vi "UHR-Fleezers Control (host) - 12.8.1.vi"() -> ()   [LabVIEW 2012] (continued)
                                n2135 = Greater?(x=w3246, y=70.0) -> (0:w3244:bool)
                                n2136 = property on="Remove Action Offset" class="Bool (strict)"("Val(Sgnl)"=w3244) -> ()  [unwired: 2 in, 2 out]
                                }
                                }
                                }
                                }
                                frame #4 {
                                n2137 = Wait (ms)(milliseconds to wait=u32 500) -> ()  [unwired: 1 out]
                                }
                                frame #5 {
                                n2138 = local read "Mean"() -> (w3255:dbl)
                                n2139 = Greater?(x=w3255, y=11.0) -> (0:w3249:bool)
                                n2140 = Not(x=w3249) -> (.not. x?=w3250:bool)
                                n2141 = And(x=w3250, y="Shift confocal") -> (x .and. y?=w3252:bool)
                                n2142 = And(x=w3249, y="Shift confocal") -> (x .and. y?=w3253:bool)
                                n2143 = case shown="True" w3253 {
                                frame False {
                                }
                                frame True {
                                n2144 = local read "Confocal Y 2 (V)"() -> (w3259:dbl)
                                n2145 = local read "Confocal X 2 (V)"() -> (w3258:dbl)
                                n2146 = property on="AO1" class="Slide (strict)"("Val(Sgnl)"=w3259) -> ()  [unwired: 2 in, 2 out]
                                n2147 = property on="AO2" class="Slide (strict)"("Val(Sgnl)"=w3258) -> ()  [unwired: 2 in, 2 out]
                                }
                                }
                                n2148 = case shown="True" w3252 {
                                frame False {
                                }
                                frame True {
                                n2149 = local read "Confocal Y 1 (V)"() -> (w3257:dbl)
                                n2150 = local read "Confocal X 1 (V)"() -> (w3256:dbl)
                                n2151 = property on="AO1" class="Slide (strict)"("Val(Sgnl)"=w3257) -> ()  [unwired: 2 in, 2 out]
                                n2152 = property on="AO2" class="Slide (strict)"("Val(Sgnl)"=w3256) -> ()  [unwired: 2 in, 2 out]
                                }
                                }
                                }
                                frame #6 {
                                n2153 = Wait (ms)(milliseconds to wait=u32 1500) -> ()  [unwired: 1 out]
                                }
                                frame #7 {
                                n2154 = property on="Rem fb disp offset" class="Bool (strict)"("Val(Sgnl)"=TRUE ("Value (Signaling)")) -> ()  [unwired: 2 in, 2 out]
                                }
                                }
                                }
                                frame True {
                                n2155 = flat-sequence {
                                tunnel: w3262 -> [w3263]
                                frame #0 {
                                n2156 = property on="Trap Delta (MHz)" class="DigNum (strict)"("Val(Sgnl)"=w3263) -> ()  [unwired: 2 in, 2 out]
                                }
                                frame #1 {
                                n2157 = Wait (ms)(milliseconds to wait=u32 500) -> ()  [unwired: 1 out]
                                }
                                frame #2 {
                                n2158 = local read "Shift confocal"() -> (w3269:bool)
                                n2159 = local read "Mean"() -> (w3271:dbl)
                                n2160 = Greater?(x=w3271, y=11.0) -> (0:w3268:bool)
                                n2161 = Not(x=w3268) -> (.not. x?=w3267:bool)
                                n2162 = And(x=w3267, y=w3269) -> (x .and. y?=w3265:bool)
                                n2163 = And(x=w3268, y=w3269) -> (x .and. y?=w3266:bool)
                                n2164 = case shown="True" w3266 {
                                frame False {
                                }
                                frame True {
                                n2165 = local read "Confocal Y 2 (V)"() -> (w3275:dbl)
                                n2166 = local read "Confocal X 2 (V)"() -> (w3274:dbl)
                                n2167 = property on="AO2" class="Slide (strict)"("Val(Sgnl)"=w3274) -> ()  [unwired: 2 in, 2 out]
                                n2168 = property on="AO1" class="Slide (strict)"("Val(Sgnl)"=w3275) -> ()  [unwired: 2 in, 2 out]
                                }
                                }
                                n2169 = case shown="True" w3265 {
                                frame False {
                                }
                                frame True {
                                n2170 = local read "Confocal X 1 (V)"() -> (w3272:dbl)
                                n2171 = local read "Confocal Y 1 (V)"() -> (w3273:dbl)
                                n2172 = property on="AO2" class="Slide (strict)"("Val(Sgnl)"=w3272) -> ()  [unwired: 2 in, 2 out]
                                n2173 = property on="AO1" class="Slide (strict)"("Val(Sgnl)"=w3273) -> ()  [unwired: 2 in, 2 out]
                                }
                                }
                                }
                                }
                                }
                                }
                                }
                                }
                                }
                                frame "Image" {
                                n2174 = property on="Confocal Image" class="Bool (strict)"("Val(Sgnl)"=TRUE ("Value (Signaling)")) -> ()  [unwired: 2 in, 2 out]
                                }
                              }
                              n2175 = local write "Fl. High"(FALSE ("Fl. High")) -> ()
                              n2176 = local read "Time (s)"() -> (w3209:dbl)
                            }
                            frame #1 {
                              n2177 = case shown="True" "Auto F Reset" {
                                tunnel: w3281 -> [_ w3286]
                                tunnel: w3280 -> [_ w3285]
                                tunnel: w3279 -> [_ w3284]
                                tunnel: w3278 -> [_ w3283]
                                frame False {
                                }
                                frame True {
                                n2178 = node-c288() -> (w3288:T27)  [unwired: 4 in]
                                n2179 = timed-loop {
                                timing: w3288 -> [_]
                                timing-out: [_] -> w3287
                                tunnel: w3286 -> [w3293]
                                tunnel: w3285 -> [w3292]
                                tunnel: w3284 -> [w3291]
                                tunnel: w3283 -> [w3290]
                                stop <- w3289 stop-if-true
                                n2180 = node-c288() -> ()  [unwired: 1 in, 1 out]
                                n2181 = local read "Fl. Delta Thresh. (kHz)"() -> (w3302:dbl)
                                n2182 = local read "APD to Watch"() -> (w3303:bool)
                                n2183 = local read "Delta Fl. 1"() -> (w3304:dbl)
                                n2184 = local read "Delta Fl. 2"() -> (w3305:dbl)
                                n2185 = local read "Fl. Triggered..."() -> (w3296:bool)
                                n2186 = local read "Stop All"() -> (w3297:bool)
                                n2187 = local read "Reset Force"() -> (w3295:bool)
                                n2188 = Multiply(x=w3302, y=1000.0) -> (x*y=w3300:dbl)
                                n2189 = Select(t=w3304, s=w3303, f=w3305) -> (s? t:f=w3299:dbl)
                                n2190 = Not(x=w3296) -> (.not. x?=w3294:bool)
                                n2191 = Greater?(x=w3299, y=w3300) -> (0:w3298:bool)
                                n2192 = Compound Arithmetic op=OR(w3298, w3297, w3294, w3295) -> (w3289:bool)
                                n2193 = case shown="True" w3289 {
                                tunnel: w3293 -> [_ w3309]
                                tunnel: w3292 -> [_ w3313]
                                tunnel: w3291 -> [_ w3312]
                                tunnel: w3290 -> [_ w3311]
                                frame False {
                                }
                                frame True {
                                n2194 = case shown="\"Yank\"" w3313 {
                                tunnel: w3312 -> [_ w3323]
                                tunnel: w3311 -> [_ w3321]
                                frame "Image", Default {
                                }
                                frame "Yank" {
                                n2195 = flat-sequence {
                                tunnel: [w3326] -> w3324
                                tunnel: w3323 -> [w3326]
                                tunnel: [w3325] -> w3322
                                tunnel: w3321 -> [w3325]
                                tunnel: w3324 -> [w3332]
                                tunnel: w3322 -> [w3330]
                                frame #0 {
                                n2196 = local read "Yank Delay (s)"() -> (w3329:dbl)
                                n2197 = Multiply(x=w3329, y=1000.0) -> (x*y=w3327:dbl)
                                n2198 = Wait (ms)(milliseconds to wait=w3327) -> ()  [unwired: 1 out]
                                }
                                frame #1 {
                                n2199 = local read "Yank to which?"() -> (w3331:bool)
                                n2200 = case shown="False" w3331 {
                                tunnel: w3332 -> [_ w3360]
                                tunnel: w3330 -> [w3333 _]
                                frame False {
                                n2201 = flat-sequence {
                                tunnel: w3333 -> [w3334]
                                frame #0 {
                                n2202 = property on="Trap Pos FB SP" class="DigNum (strict)"("Val(Sgnl)"=w3334) -> ()  [unwired: 2 in, 2 out]
                                }
                                frame #1 {
                                n2203 = Wait (ms)(milliseconds to wait=u32 700) -> ()  [unwired: 1 out]
                                }
                                frame #2 {
                                n2204 = local read "Action (%)"() -> (w3339:dbl)
                                n2205 = Absolute Value(x=w3339) -> (abs(x)=w3338:dbl)
                                n2206 = Greater?(x=w3338, y=70.0) -> (0:w3336:bool)
                                n2207 = property on="Remove Action Offset" class="Bool (strict)"("Val(Sgnl)"=w3336) -> ()  [unwired: 2 in, 2 out]
                                }
                                frame #3 {
                                n2208 = for {
                                N: 4 -> [_]
                                n2209 = flat-sequence {
                                frame #0 {
                                n2210 = Wait (ms)(milliseconds to wait=u32 500) -> ()  [unwired: 1 out]
                                }
                                frame #1 {
                                n2211 = local read "Action (%)"() -> (w3345:dbl)
                                n2212 = Absolute Value(x=w3345) -> (abs(x)=w3344:dbl)
                                n2213 = Greater?(x=w3344, y=70.0) -> (0:w3342:bool)
                                n2214 = property on="Remove Action Offset" class="Bool (strict)"("Val(Sgnl)"=w3342) -> ()  [unwired: 2 in, 2 out]
                                }
                                }
                                }
                                }
                                frame #4 {
                                n2215 = Wait (ms)(milliseconds to wait=u32 500) -> ()  [unwired: 1 out]
                                }
                                frame #5 {
                                n2216 = local read "Shift confocal"() -> (w3350:bool)
                                n2217 = local read "Mean"() -> (w3353:dbl)
                                n2218 = Greater?(x=w3353, y=11.0) -> (0:w3349:bool)
                                n2219 = Not(x=w3349) -> (.not. x?=w3348:bool)
                                n2220 = And(x=w3349, y=w3350) -> (x .and. y?=w3351:bool)
                                n2221 = And(x=w3348, y=w3350) -> (x .and. y?=w3347:bool)
                                n2222 = case shown="True" w3351 {
                                frame False {
                                }
                                frame True {
                                n2223 = local read "Confocal X 2 (V)"() -> (w3356:dbl)
                                n2224 = local read "Confocal Y 2 (V)"() -> (w3357:dbl)
                                n2225 = property on="AO2" class="Slide (strict)"("Val(Sgnl)"=w3356) -> ()  [unwired: 2 in, 2 out]
                                n2226 = property on="AO1" class="Slide (strict)"("Val(Sgnl)"=w3357) -> ()  [unwired: 2 in, 2 out]
                                }
                                }
                                n2227 = case shown="True" w3347 {
                                frame False {
                                }
                                frame True {
                                n2228 = local read "Confocal Y 1 (V)"() -> (w3355:dbl)
                                n2229 = local read "Confocal X 1 (V)"() -> (w3354:dbl)
                                n2230 = property on="AO1" class="Slide (strict)"("Val(Sgnl)"=w3355) -> ()  [unwired: 2 in, 2 out]
                                n2231 = property on="AO2" class="Slide (strict)"("Val(Sgnl)"=w3354) -> ()  [unwired: 2 in, 2 out]
                                }
                                }
                                }
                                frame #6 {
                                n2232 = Wait (ms)(milliseconds to wait=u32 1500) -> ()  [unwired: 1 out]
                                }
                                frame #7 {
                                n2233 = property on="Rem fb disp offset" class="Bool (strict)"("Val(Sgnl)"=TRUE ("Value (Signaling)")) -> ()  [unwired: 2 in, 2 out]
                                }
                                }
                                }
                                frame True {
                                n2234 = flat-sequence {
                                tunnel: w3360 -> [w3361]
                                frame #0 {
                                n2235 = property on="Trap Delta (MHz)" class="DigNum (strict)"("Val(Sgnl)"=w3361) -> ()  [unwired: 2 in, 2 out]
                                }
                                frame #1 {
                                n2236 = Wait (ms)(milliseconds to wait=u32 500) -> ()  [unwired: 1 out]
                                }
                                frame #2 {
                                n2237 = local read "Shift confocal"() -> (w3367:bool)
                                n2238 = local read "Mean"() -> (w3368:dbl)
                                n2239 = Greater?(x=w3368, y=11.0) -> (0:w3366:bool)
                                n2240 = And(x=w3366, y=w3367) -> (x .and. y?=w3364:bool)
                                n2241 = Not(x=w3366) -> (.not. x?=w3365:bool)
                                n2242 = And(x=w3365, y=w3367) -> (x .and. y?=w3363:bool)
                                n2243 = case shown="True" w3364 {
                                frame False {
                                }
                                frame True {
                                n2244 = local read "Confocal Y 2 (V)"() -> (w3373:dbl)
                                n2245 = local read "Confocal X 2 (V)"() -> (w3372:dbl)
                                n2246 = property on="AO1" class="Slide (strict)"("Val(Sgnl)"=w3373) -> ()  [unwired: 2 in, 2 out]
                                n2247 = property on="AO2" class="Slide (strict)"("Val(Sgnl)"=w3372) -> ()  [unwired: 2 in, 2 out]
                                }
                                }
                                n2248 = case shown="True" w3363 {
                                frame False {
                                }
                                frame True {
                                n2249 = local read "Confocal Y 1 (V)"() -> (w3371:dbl)
                                n2250 = local read "Confocal X 1 (V)"() -> (w3370:dbl)
                                n2251 = property on="AO2" class="Slide (strict)"("Val(Sgnl)"=w3370) -> ()  [unwired: 2 in, 2 out]
                                n2252 = property on="AO1" class="Slide (strict)"("Val(Sgnl)"=w3371) -> ()  [unwired: 2 in, 2 out]
                                }
                                }
                                }
                                }
                                }
                                }
                                }
                                }
                                }
                                }
                                n2253 = local read "Time (s)"() -> (w3308:dbl)
                                n2254 = Subtract(x=w3309, y=w3308) -> (x-y=w3320:dbl)
                                n2255 = Number To Decimal String(number=w3320, width (-)=i16 0) -> (decimal integer string=w3318:string)
                                n2256 = Concatenate Strings(w3318, " s fluorescence event") -> (w3315:string)
                                n2257 = local read "Messages"() -> (w3316:string)
                                n2258 = local write "Duration (s)"(w3320) -> ()
                                n2259 = call "Update messages.vi"("Message to add"=w3315, "Old message string"=w3316) -> ("New message string"=w3314:string)
                                n2260 = local write "Messages"(w3314) -> ()
                                n2261 = call <vilib>:"Beep.vi"() -> ()  [unwired: 12 in]
                                n2262 = local write "Reset Force"(FALSE ("Force Reset")) -> ()
                                n2263 = local write "Fl. High"(TRUE ("Fl. High")) -> ()
                                n2264 = local write "Waiting"(TRUE ("Waiting")) -> ()
                                }
                                }
                                n2265 = node-c288() -> ()  [unwired: 1 in, 1 out]
                                }
                                n2266 = node-c288(w3287) -> ()  [unwired: 1 out]
                                }
                              }
                            }
                          }
                          n2267 = local read "Trap Delta (MHz)"() -> (w3199:dbl)
                          n2268 = local read "Trap Pos FB SP"() -> (w3197:fxp<+/-,16,1>)
                        }
                      }
                    }
                    frame True {
                      n2269 = flat-sequence {
                        tunnel: w3384 -> [w3394]
                        tunnel: [w3394] -> w3388
                        tunnel: w3387 -> [w3393]
                        tunnel: [w3393] -> w3386
                        tunnel: [w3392] -> w3385
                        tunnel: w3383 -> [w3391]
                        tunnel: [w3390] -> w3382
                        tunnel: w3379 -> [w3389]
                        tunnel: [w3389] -> w3378
                        tunnel: w3388 -> [w3464]
                        tunnel: w3386 -> [w3463]
                        tunnel: w3385 -> [w3462]
                        tunnel: w3382 -> [w3461]
                        tunnel: w3378 -> [w3460]
                        tunnel: [w3461] -> w3381
                        frame #0 {
                          n2270 = call <vilib>:"Beep.vi"() -> ()  [unwired: 3 in, 9 out]
                          n2271 = local write "Waiting"(FALSE ("Waiting")) -> ()
                          n2272 = Increment(x=w3391) -> (x+1=w3390:u8)
                          n2273 = case shown="\"Yank\"" w3393 {
                            tunnel: w3390 -> [_ _ w3400]
                            frame "Image" {
                              n2274 = property on="Confocal Image" class="Bool (strict)"("Val(Sgnl)"=TRUE ("Value (Signaling)")) -> ()  [unwired: 2 in, 2 out]
                            }
                            frame "Alarm", Default {
                            }
                            frame "Yank" {
                              n2275 = flat-sequence {
                                tunnel: w3400 -> [w3403]
                                tunnel: [w3402] -> w3399
                                tunnel: ["N Array El"] -> w3398
                                tunnel: w3399 -> [w3417]
                                tunnel: w3398 -> [w3413]
                                frame #0 {
                                n2276 = Multiply(x="Yank Delay (s)", y=1000.0) -> (x*y=w3406:dbl)
                                n2277 = Quotient & Remainder(x=w3403, y="N Array El") -> (x-y*floor(x/y)=w3402:u8)  [unwired: 1 out]
                                n2278 = Wait (ms)(milliseconds to wait=w3406) -> ()  [unwired: 1 out]
                                }
                                frame #1 {
                                n2279 = Random Number (0-1)() -> (number: 0 to 1=w3414:dbl)
                                n2280 = Multiply(x=w3413, y=w3414) -> (x*y=w3412:dbl)
                                n2281 = Round Toward -Infinity(1:w3412) -> (0:w3411:dbl)
                                n2282 = Select(t=w3411, s="Random Choice", f=w3417) -> (s? t:f=w3415:dbl)
                                n2283 = Select(t="Yank to Trap Delta (MHz)", s="Yank to which?", f="Yank to SP") -> (s? t:f=w3408:dbl[])
                                n2284 = Index Array(array=w3408, index=w3415) -> (element=w3418:dbl)
                                n2285 = case shown="False" "Yank to which?" {
                                tunnel: w3418 -> [w3419 w3445]
                                frame False {
                                n2286 = flat-sequence {
                                tunnel: w3419 -> [w3420]
                                frame #0 {
                                n2287 = property on="Trap Pos FB SP" class="DigNum (strict)"("Val(Sgnl)"=w3420) -> ()  [unwired: 2 in, 2 out]
                                }
                                frame #1 {
                                n2288 = Wait (ms)(milliseconds to wait=u32 700) -> ()  [unwired: 1 out]
                                }
                                frame #2 {
                                n2289 = local read "Action (%)"() -> (w3425:dbl)
                                n2290 = Absolute Value(x=w3425) -> (abs(x)=w3424:dbl)
                                n2291 = Greater?(x=w3424, y=70.0) -> (0:w3422:bool)
                                n2292 = property on="Remove Action Offset" class="Bool (strict)"("Val(Sgnl)"=w3422) -> ()  [unwired: 2 in, 2 out]
                                }
                                frame #3 {
                                n2293 = for {
                                N: 4 -> [_]
                                n2294 = flat-sequence {
                                frame #0 {
                                n2295 = Wait (ms)(milliseconds to wait=u32 500) -> ()  [unwired: 1 out]
                                }
                                frame #1 {
                                n2296 = local read "Action (%)"() -> (w3431:dbl)
                                n2297 = Absolute Value(x=w3431) -> (abs(x)=w3430:dbl)
                                n2298 = Greater?(x=w3430, y=70.0) -> (0:w3428:bool)
                                n2299 = property on="Remove Action Offset" class="Bool (strict)"("Val(Sgnl)"=w3428) -> ()  [unwired: 2 in, 2 out]
                                }
                                }
                                }
                                }
                                frame #4 {
                                n2300 = local read "Shift confocal"() -> (w3435:bool)
                                n2301 = local read "Mean"() -> (w3438:dbl)
                                n2302 = Greater?(x=w3438, y=11.0) -> (0:w3434:bool)
                                n2303 = Not(x=w3434) -> (.not. x?=w3433:bool)
                                n2304 = And(x=w3433, y=w3435) -> (x .and. y?=w3432:bool)
                                n2305 = And(x=w3434, y=w3435) -> (x .and. y?=w3436:bool)
                                n2306 = case shown="True" w3436 {
                                frame False {
                                }
                                frame True {
                                n2307 = local read "Confocal X 2 (V)"() -> (w3441:dbl)
                                n2308 = local read "Confocal Y 2 (V)"() -> (w3442:dbl)
                                n2309 = property on="AO2" class="Slide (strict)"("Val(Sgnl)"=w3441) -> ()  [unwired: 2 in, 2 out]
                                n2310 = property on="AO1" class="Slide (strict)"("Val(Sgnl)"=w3442) -> ()  [unwired: 2 in, 2 out]
                                }
                                }
                                n2311 = case shown="True" w3432 {
                                frame False {
                                }
                                frame True {
                                n2312 = local read "Confocal X 1 (V)"() -> (w3439:dbl)
                                n2313 = local read "Confocal Y 1 (V)"() -> (w3440:dbl)
                                n2314 = property on="AO1" class="Slide (strict)"("Val(Sgnl)"=w3440) -> ()  [unwired: 2 in, 2 out]
                                n2315 = property on="AO2" class="Slide (strict)"("Val(Sgnl)"=w3439) -> ()  [unwired: 2 in, 2 out]
                                }
                                }
                                }
                                frame #5 {
                                n2316 = Wait (ms)(milliseconds to wait=u32 1500) -> ()  [unwired: 1 out]
                                }
                                frame #6 {
                                n2317 = property on="Rem fb disp offset" class="Bool (strict)"("Val(Sgnl)"=TRUE ("Value (Signaling)")) -> ()  [unwired: 2 in, 2 out]
                                }
                                }
                                }
                                frame True {
                                n2318 = flat-sequence {
                                tunnel: w3445 -> [w3446]
                                frame #0 {
                                n2319 = property on="Trap Delta (MHz)" class="DigNum (strict)"("Val(Sgnl)"=w3446) -> ()  [unwired: 2 in, 2 out]
                                }
                                frame #1 {
                                n2320 = Wait (ms)(milliseconds to wait=u32 500) -> ()  [unwired: 1 out]
                                }
                                frame #2 {
                                n2321 = local read "Shift confocal"() -> (w3450:bool)
                                n2322 = local read "Mean"() -> (w3448:dbl)
                                n2323 = Greater?(x=w3448, y=11.0) -> (0:w3451:bool)
                                n2324 = Not(x=w3451) -> (.not. x?=w3452:bool)
                                n2325 = And(x=w3452, y=w3450) -> (x .and. y?=w3454:bool)
                                n2326 = And(x=w3451, y=w3450) -> (x .and. y?=w3453:bool)
                                n2327 = case shown="True" w3453 {
                                frame False {
                                }
                                frame True {
                                n2328 = local read "Confocal Y 2 (V)"() -> (w3458:dbl)
                                n2329 = local read "Confocal X 2 (V)"() -> (w3457:dbl)
                                n2330 = property on="AO1" class="Slide (strict)"("Val(Sgnl)"=w3458) -> ()  [unwired: 2 in, 2 out]
                                n2331 = property on="AO2" class="Slide (strict)"("Val(Sgnl)"=w3457) -> ()  [unwired: 2 in, 2 out]
                                }
                                }
                                n2332 = case shown="True" w3454 {
                                frame False {
                                }
                                frame True {
                                n2333 = local read "Confocal X 1 (V)"() -> (w3455:dbl)
                                n2334 = local read "Confocal Y 1 (V)"() -> (w3456:dbl)
                                n2335 = property on="AO2" class="Slide (strict)"("Val(Sgnl)"=w3455) -> ()  [unwired: 2 in, 2 out]
                                n2336 = property on="AO1" class="Slide (strict)"("Val(Sgnl)"=w3456) -> ()  [unwired: 2 in, 2 out]
                                }
                                }
                                }
                                }
                                }
                                }
                                }
                              }
                            }
                          }
                          n2337 = local read "Time (s)"() -> (w3392:dbl)
                          "Fl. High" <- TRUE ("Yanking")
                        }
                        frame #1 {
                          n2338 = local read "Auto F Reset"() -> (w3459:bool)
                          n2339 = case shown="True" w3459 {
                            tunnel: w3464 -> [_ w3468]
                            tunnel: w3463 -> [_ w3467]
                            tunnel: w3462 -> [_ w3466]
                            tunnel: w3460 -> [_ w3465]
                            frame False {
                            }
                            frame True {
                              n2340 = node-c288() -> (w3470:T27)  [unwired: 4 out]
                              n2341 = timed-loop {
                                timing: w3470 -> [_]
                                timing-out: [_] -> w3469
                                tunnel: w3468 -> [w3488]
                                tunnel: w3467 -> [w3487]
                                tunnel: w3466 -> [w3486]
                                tunnel: w3465 -> [w3485]
                                stop <- w3471 stop-if-true
                                n2342 = node-c288() -> ()  [unwired: 2 out]
                                n2343 = local read "Fl. Delta Thresh. (kHz)"() -> (w3479:dbl)
                                n2344 = local read "Fl. Triggered..."() -> (w3484:bool)
                                n2345 = local read "Delta Fl. 1"() -> (w3475:dbl)
                                n2346 = local read "Delta Fl. 2"() -> (w3473:dbl)
                                n2347 = local read "Stop All"() -> (w3482:bool)
                                n2348 = local read "APD to Watch"() -> (w3474:bool)
                                n2349 = Select(t=w3475, s=w3474, f=w3473) -> (s? t:f=w3472:dbl)
                                n2350 = Not(x=w3484) -> (.not. x?=w3483:bool)
                                n2351 = Multiply(x=w3479, y=1000.0) -> (x*y=w3478:dbl)
                                n2352 = Negate(x=w3478) -> (-x=w3477:dbl)
                                n2353 = Less?(x=w3472, y=w3477) -> (x < y?=w3481:bool)
                                n2354 = Compound Arithmetic op=OR(w3481, w3482, w3483, "Reset Force") -> (w3471:bool)
                                n2355 = case shown="True" w3471 {
                                tunnel: w3488 -> [_ w3503]
                                tunnel: w3487 -> [_ w3502]
                                tunnel: w3486 -> [_ w3492]
                                tunnel: w3485 -> [_ w3494]
                                frame False {
                                }
                                frame True {
                                n2356 = local read "Time (s)"() -> (w3493:dbl)
                                n2357 = case shown="\"Yank\"" w3502 {
                                tunnel: w3503 -> [_ w3506]
                                tunnel: w3494 -> [_ w3504]
                                frame "Image", Default {
                                }
                                frame "Yank" {
                                n2358 = flat-sequence {
                                tunnel: [w3512] -> w3507
                                tunnel: w3506 -> [w3512]
                                tunnel: [w3508] -> w3505
                                tunnel: w3504 -> [w3508]
                                tunnel: w3507 -> [w3515]
                                tunnel: w3505 -> [w3513]
                                frame #0 {
                                n2359 = local read "Yank Delay (s)"() -> (w3511:dbl)
                                n2360 = Multiply(x=w3511, y=1000.0) -> (x*y=w3509:dbl)
                                n2361 = Wait (ms)(milliseconds to wait=w3509) -> ()  [unwired: 1 out]
                                }
                                frame #1 {
                                n2362 = local read "Yank to which?"() -> (w3514:bool)
                                n2363 = case shown="False" w3514 {
                                tunnel: w3515 -> [_ w3542]
                                tunnel: w3513 -> [w3516 _]
                                frame False {
                                n2364 = flat-sequence {
                                tunnel: w3516 -> [w3517]
                                frame #0 {
                                n2365 = property on="Trap Pos FB SP" class="DigNum (strict)"("Val(Sgnl)"=w3517) -> ()  [unwired: 2 in, 2 out]
                                }
                                frame #1 {
                                n2366 = Wait (ms)(milliseconds to wait=u32 700) -> ()  [unwired: 1 out]
                                }
                                frame #2 {
                                n2367 = local read "Action (%)"() -> (w3522:dbl)
                                n2368 = Absolute Value(x=w3522) -> (abs(x)=w3521:dbl)
                                n2369 = Greater?(x=w3521, y=70.0) -> (0:w3519:bool)
                                n2370 = property on="Remove Action Offset" class="Bool (strict)"("Val(Sgnl)"=w3519) -> ()  [unwired: 2 in, 2 out]
                                }
                                frame #3 {
                                n2371 = for {
                                N: 4 -> [_]
                                n2372 = flat-sequence {
                                frame #0 {
                                n2373 = Wait (ms)(milliseconds to wait=u32 500) -> ()  [unwired: 1 out]
                                }
                                frame #1 {
                                n2374 = local read "Action (%)"() -> (w3528:dbl)
                                n2375 = Absolute Value(x=w3528) -> (abs(x)=w3527:dbl)
                                n2376 = Greater?(x=w3527, y=70.0) -> (0:w3525:bool)
                                n2377 = property on="Remove Action Offset" class="Bool (strict)"("Val(Sgnl)"=w3525) -> ()  [unwired: 2 in, 2 out]
                                }
                                }
                                }
                                }
                                frame #4 {
                                n2378 = local read "Shift confocal"() -> (w3533:bool)
                                n2379 = local read "Mean"() -> (w3535:dbl)
                                n2380 = Greater?(x=w3535, y=11.0) -> (0:w3532:bool)
                                n2381 = Not(x=w3532) -> (.not. x?=w3531:bool)
                                n2382 = And(x=w3532, y=w3533) -> (x .and. y?=w3530:bool)
                                n2383 = And(x=w3531, y=w3533) -> (x .and. y?=w3529:bool)
                                n2384 = case shown="True" w3530 {
                                frame False {
                                }
                                frame True {
                                n2385 = local read "Confocal Y 2 (V)"() -> (w3539:dbl)
                                n2386 = local read "Confocal X 2 (V)"() -> (w3538:dbl)
                                n2387 = property on="AO2" class="Slide (strict)"("Val(Sgnl)"=w3538) -> ()  [unwired: 2 in, 2 out]
                                n2388 = property on="AO1" class="Slide (strict)"("Val(Sgnl)"=w3539) -> ()  [unwired: 2 in, 2 out]
                                }
                                }
                                n2389 = case shown="True" w3529 {
                                frame False {
                                }
                                frame True {
                                n2390 = local read "Confocal X 1 (V)"() -> (w3536:dbl)
                                n2391 = local read "Confocal Y 1 (V)"() -> (w3537:dbl)
                                n2392 = property on="AO1" class="Slide (strict)"("Val(Sgnl)"=w3537) -> ()  [unwired: 2 in, 2 out]
                                n2393 = property on="AO2" class="Slide (strict)"("Val(Sgnl)"=w3536) -> ()  [unwired: 2 in, 2 out]
                                }
                                }
                                }
                                frame #5 {
                                n2394 = Wait (ms)(milliseconds to wait=u32 1500) -> ()  [unwired: 1 out]
                                }
                                frame #6 {
                                n2395 = property on="Rem fb disp offset" class="Bool (strict)"("Val(Sgnl)"=TRUE ("Value (Signaling)")) -> ()  [unwired: 2 in, 2 out]
                                }
                                }
                                }
                                frame True {
                                n2396 = flat-sequence {
                                tunnel: w3542 -> [w3543]
                                frame #0 {
                                n2397 = property on="Trap Delta (MHz)" class="DigNum (strict)"("Val(Sgnl)"=w3543) -> ()  [unwired: 2 in, 2 out]
                                }
                                frame #1 {
                                n2398 = Wait (ms)(milliseconds to wait=u32 500) -> ()  [unwired: 1 out]
                                }
                                frame #2 {
                                n2399 = local read "Shift confocal"() -> (w3549:bool)
                                n2400 = local read "Mean"() -> (w3551:dbl)
                                n2401 = Greater?(x=w3551, y=11.0) -> (0:w3548:bool)
                                n2402 = Not(x=w3548) -> (.not. x?=w3547:bool)
                                n2403 = And(x=w3548, y=w3549) -> (x .and. y?=w3546:bool)
                                n2404 = And(x=w3547, y=w3549) -> (x .and. y?=w3545:bool)
                                n2405 = case shown="True" w3546 {
                                frame False {
                                }
                                frame True {
                                n2406 = local read "Confocal Y 2 (V)"() -> (w3555:dbl)
                                n2407 = local read "Confocal X 2 (V)"() -> (w3554:dbl)
                                n2408 = property on="AO2" class="Slide (strict)"("Val(Sgnl)"=w3554) -> ()  [unwired: 2 in, 2 out]
                                n2409 = property on="AO1" class="Slide (strict)"("Val(Sgnl)"=w3555) -> ()  [unwired: 2 in, 2 out]
                                }
                                }
                                n2410 = case shown="True" w3545 {
                                frame False {
                                }
                                frame True {
                                n2411 = local read "Confocal Y 1 (V)"() -> (w3553:dbl)
                                n2412 = local read "Confocal X 1 (V)"() -> (w3552:dbl)
                                n2413 = property on="AO2" class="Slide (strict)"("Val(Sgnl)"=w3552) -> ()  [unwired: 2 in, 2 out]
                                n2414 = property on="AO1" class="Slide (strict)"("Val(Sgnl)"=w3553) -> ()  [unwired: 2 in, 2 out]
                                }
                                }
                                }
                                }
                                }
                                }
                                }
                                }
                                }
                                }
                                n2415 = local read "Messages"() -> (w3501:string)
                                n2416 = Subtract(x=w3493, y=w3492) -> (x-y=w3499:dbl)
                                "Duration (s)" <- w3499
                                n2417 = Number To Decimal String(number=w3499, width (-)=i16 0) -> (decimal integer string=w3497:string)
                                n2418 = Concatenate Strings(w3497, " s fluorescence event." ("string")) -> (w3495:string)
                                n2419 = call "Update messages.vi"("Message to add"=w3495, "Old message string"=w3501) -> ("New message string"=w3500:string)
                                n2420 = local write "Reset Force"(FALSE ("Reset Force")) -> ()
                                n2421 = local write "Waiting"(TRUE ("Waiting")) -> ()
                                n2422 = local write "Messages"(w3500) -> ()
                                n2423 = local write "Fl. High"(FALSE ("Fl. High")) -> ()
                                n2424 = call <vilib>:"Beep.vi"() -> ()  [unwired: 3 in, 9 out]
                                }
                                }
                                n2425 = node-c288() -> ()  [unwired: 2 out]
                              }
                              n2426 = node-c288(w3469) -> ()  [unwired: 1 out]
                            }
                          }
                        }
                      }
                      n2427 = local read "Trap Delta (MHz)"() -> (w3384:dbl)
                      n2428 = local read "Trap Pos FB SP"() -> (w3379:fxp<+/-,16,1>)
                    }
                  }
                }
                frame #1 {
                  n2429 = local read "Stop All"() -> (w3565:bool)
                  n2430 = local read "Fl. Triggered..."() -> (w3563:bool)
                  n2431 = Not(x=w3563) -> (.not. x?=w3564:bool)
                  n2432 = Or(x=w3564, y=w3565) -> (x .or. y?=w3562:bool)
                }
              }
              n2433 = case shown="True" w3156 {
                frame False {
                }
                frame True {
                  n2434 = local read "Confocal Y 1 (V)"() -> (w3166:dbl)
                  n2435 = local read "Confocal X 1 (V)"() -> (w3165:dbl)
                  n2436 = property on="AO2" class="Slide (strict)"("Val(Sgnl)"=w3165) -> ()  [unwired: 2 in, 2 out]
                  n2437 = property on="AO1" class="Slide (strict)"("Val(Sgnl)"=w3166) -> ()  [unwired: 2 in, 2 out]
                }
              }
              n2438 = case shown="True" w3156 {
                frame False {
                }
                frame True {
                  w3164 = FALSE ("Fl. High")
                  n2439 = local write "Waiting"(w3164) -> ()
                  n2440 = local write "Fl. High"(w3164) -> ()
                }
              }
              n2441 = node-c288() -> ()  [unwired: 2 out]
            }
            n2442 = node-c288(w3154) -> ()  [unwired: 1 out]
          }
        }
      }
      event "Stop All": Value Change {
        n2443 = event-data() -> ()  [unwired: 7 out]
        n2444 = local read "Stop All"() -> (w3570:bool)
      }
    }
    n2445 = node-c288() -> ()  [unwired: 2 out]
  }
  n2446 = node-c288(i64 1 ("Period"), 1 ("Processor")) -> (w85:T27)  [unwired: 2 out]
  n2447 = node-c288(w33) -> ()  [unwired: 1 out]
  n2448 = node-c288(w77) -> ()  [unwired: 1 out]
  n2449 = node-c288(w79) -> ()  [unwired: 1 out]
  n2450 = property on="Saved trap pos" class="WFGraph (strict)"("Visible"=FALSE) -> ()  [unwired: 2 in, 2 out]
  n2451 = property on="Trap Delta Graph" class="WFGraph (strict)"("Visible"=TRUE) -> ()  [unwired: 2 in, 2 out]
  n2452 = node-c288(w65) -> ()  [unwired: 1 out]
  n2453 = local write "Trap pos"(FALSE ("Trap pos")) -> ()
  n2454 = Unbundle By Name("sound format") -> ("sample rate (S/s)"=w4:dbl)
  n2455 = call <vilib>:"Sound Output Configure.vi"("number of samples/ch"="number of samples/ch", "sample mode"="sample mode", "sound format"="sound format", "device ID"="device ID") -> ("task ID"=w8:T42)  [unwired: 6 in, 1 out]
  n2456 = local read "DMA Update Period (s)"() -> (w5:dbl)
  n2457 = Multiply(x=w5, y=w4) -> (x*y=w3:dbl)
  n2458 = for "Sound time base" {
    N: w3 -> [_]
    tunnel: [w3571] -> w6 mode=indexing
    i -> [w3571]
  }
  n2459 = Reciprocal(x=w4) -> (1/x=w2:dbl)
  n2460 = Multiply(x=w6, y=w2) -> (x*y=w1:dbl[])
  n2461 = timed-loop "Main data acquisition loop (get data, process data for display, and save data to disk)" {
    tunnel: w23 -> [w3887]
    tunnel: w22 -> [w3886]
    tunnel: [w3915] -> w92
    tunnel: [w3910] -> w91
    timing: w85 -> [_]
    timing-out: [_] -> w84
    tunnel: w59 -> [w3771]
    tunnel: [w3597] -> w12
    tunnel: w8 -> [w3596]
    tunnel: w4 -> [w3594]
    tunnel: w3 -> [w3593]
    tunnel: w2 -> [w3592]
    tunnel: w1 -> [w3591]
    stop <- "Stop All" stop-if-true
    w3688 = "Initialize"
    # "List of channels in order (X or Y only):\nT1 X (mV)\nT2 X (mV)\nT1 X (nm)\nT2 X (nm)\nT1 FX (pN)\nT2 FX (pN)\nPosition Difference (nm)\nAPD1\nAPD2\nAPD3"
    # "T2 sum"
    # "T1 sum"
    # "Fluorescence data into FIFO for external control vi's\n(e.g., fluorescence triggering) - Duncan Nall"
    n2462 = node-c288() -> ()  [unwired: 2 out]
    n2463 = First Call?() -> (First Call?: T/F=w3723:bool)
    n2464 = Or(x="Reset", y=w3723) -> (x .or. y?=w3724:bool)
    n2465 = local read "Flushing P1"() -> (w3646:bool)
    n2466 = case "Reset data stream (manual reset or at begining of some rastering and imaging)" shown="True" w3724 {
      tunnel: w3887 -> [w4970 w4978]
      tunnel: w3886 -> [w4969 w4977]
      tunnel: [w4970 w4972] -> w3882
      tunnel: [w4969 w4971] -> w3881
      frame False {
      }
      frame True {
        w4975 = TRUE ("AI to FIFO")
        n2467 = local write "Overflow (data lost)"(FALSE ("Overflow (data lost)")) -> ()
        n2468 = call "reset FPGA DMA.vi"("error in"=w4977, "FPGA VI Reference In"=w4978) -> ("error out"=w4973:errorcluster, "FPGA VI Reference Out"=w4974:T24)
        n2469 = xnode "Read/Write Control"("FPGA VI Reference In"=w4974, "error in"=w4973, "AI to FIFO"=w4975, "APD to FIFO"=w4975) -> ("FPGA VI Reference Out"=w4972:T24, "error out"=w4971:errorcluster)
      }
    }
    n2470 = case shown="True" w3646 {
      frame False {
      }
      frame True {
        n2471 = local read "Flush rate (uL/m) P1"() -> (w4005:dbl)
        n2472 = local read "HP1 Flush Time (s)"() -> (w4014:dbl)
        n2473 = local read "DMA Update Period (s)"() -> (w4008:dbl)
        n2474 = Divide(x=w4005, y=60.0) -> (x/y=w4006:dbl)
        n2475 = Divide(x=w4014, y=w4008) -> (x/y=w4003:dbl)
        n2476 = feedback #4(0) -> (w4012:i32)
        n2477 = Increment(x=w4012) -> (x+1=w4002:i32)
        n2478 = Greater?(x=w4002, y=w4003) -> (0:w4011:bool)
        n2479 = Compound Arithmetic op=MULTIPLY(w4008, w4002, w4006) -> (→"P1 Flush Volume (uL)":dbl)
        n2480 = Divide(x=w4002, y=w4003) -> (x/y=→"P1 Flushing Bar":dbl)
        n2481 = case shown="True" w4011 {
          tunnel: w4002 -> [w4015 _]
          tunnel: [w4015 0] -> w4010
          frame False {
          }
          frame True {
            w4016 = FALSE ("Flushing P1")
            n2482 = local write "Inject Pump 1"(w4016) -> ()
            n2483 = local write "Flushing P1"(w4016) -> ()
            n2484 = property on="Clear Volume P1" class="Bool (strict)"("Val(Sgnl)"=TRUE ("Value (Signaling)")) -> ()  [unwired: 2 in, 2 out]
          }
        }
        n2485 = feedback-in #4(w4010) -> ()
      }
    }
    n2486 = Or(x="Start AOD Scan", y="Trap Raster Scan") -> (x .or. y?=w3846:bool)
    n2487 = case "Start AOM raster scan" shown="True" w3846 {
      tunnel: w3882 -> [w4820 w4830]
      tunnel: w3881 -> [w4819 w4829]
      tunnel: [w4820 w4823] -> w3880
      tunnel: [w4819 w4822] -> w3879
      frame False {
      }
      frame True {
        n2488 = case shown="True" "Restart DMA? (AOD)" {
          tunnel: [w4868 w4870] -> w4824
          tunnel: [w4867 w4869] -> w4825
          tunnel: w4830 -> [w4868 w4872]
          tunnel: w4829 -> [w4867 w4871]
          frame False {
          }
          frame True {
            n2489 = local write "Overflow (data lost)"(FALSE ("Overflow (data lost)")) -> ()
            n2490 = call "reset FPGA DMA.vi"("error in"=w4871, "FPGA VI Reference In"=w4872) -> ("error out"=w4869:errorcluster, "FPGA VI Reference Out"=w4870:T24)
          }
        }
        n2491 = local write "Trap Raster Scan"(FALSE ("Trap Raster Scan")) -> ()
        n2492 = case shown="True" "Move MCL Also?" {
          tunnel: w4825 -> [w4833 w4862]
          tunnel: w4824 -> [w4834 w4863]
          tunnel: [w4832 w4866] -> w4823
          tunnel: [w4831 w4865] -> w4822
          frame False {
            w4835 = TRUE ("AI to FIFO")
            n2493 = xnode "Read/Write Control"("FPGA VI Reference In"=w4834, "error in"=w4833, "AI to FIFO"=w4835, "APD to FIFO"=w4835, "Start scan"=w4835) -> ("FPGA VI Reference Out"=w4832:T24, "error out"=w4831:errorcluster)
          }
          frame True {
            w4859 = FALSE ("1D or 2D Scan?")
            w4864 = TRUE ("AI to FIFO")
            # "Count for MCL loop"
            # "N total cycles"
            # "N steps"
            # "V_int"
            n2494 = local read "Scan Range (nm)"() -> (w4841:dbl)
            n2495 = local read "Number of F/B Scans (AOD)"() -> (w4858:u16)
            n2496 = Sign(1:w4841) -> (0:w4840:dbl)
            n2497 = Compound Arithmetic op=MULTIPLY(w4841, "MCL Step Position Ratio", "MCL/AOM Scale Tweak") -> (w4845:dbl)
            n2498 = Negate(x=w4840) -> (-x=w4837:dbl)
            n2499 = Multiply(x=w4837, y="MCL Step Increment (V_int)") -> (x*y=w4839:dbl)
            n2500 = Divide(x=w4845, y="MCL X Cal (nm/V)") -> (x/y=w4851:dbl)
            n2501 = Multiply(x=32767.0 ("y"), y=w4851) -> (x*y=w4857:dbl)
            n2502 = local read "Total Counts (ticks)"() -> (w4842:u16)
            n2503 = local read "Cycles/step (AOD)"() -> (w4853:u64)
            n2504 = local read "Scan steps (AOD)"() -> (w4854:u64)
            n2505 = Divide(x=w4857, y=10.0) -> (x/y=w4850:dbl)
            n2506 = Divide(x=w4850, y="MCL Step Increment (V_int)") -> (x/y=w4848:dbl)
            n2507 = Absolute Value(x=w4848) -> (abs(x)=w4836:dbl)
            n2508 = Compound Arithmetic op=MULTIPLY(w4854, w4853, w4842) -> (w4849:u64)
            n2509 = local write "wait to reset values"(w4864) -> ()
            n2510 = local write "MCL Scanning"(w4864) -> ()
            n2511 = Divide(x=w4849, y=w4836) -> (x/y=w4846:dbl)
            "MCL Count" <- w4846
            n2512 = xnode "Read/Write Control"("FPGA VI Reference In"=w4863, "error in"=w4862, "Scan steps (MCL)"=w4836, "Number of scans (MCL)"=w4858, "Cycles per step (MCL)"=u64 1, "Scan freq.  increment (MCL)"=w4839, "1D or 2D Scan?"=w4859, "MCL Scan Axis"=w4859, "Cont. Scan (MCL)"=w4859, "MCL count"=w4846) -> ("FPGA VI Reference Out"=w4861:T24, "error out"=w4860:errorcluster)
            n2513 = xnode "Read/Write Control"("FPGA VI Reference In"=w4861, "error in"=w4860, "AI to FIFO"=w4864, "APD to FIFO"=w4864, "Start scan"=w4864, "Start scan (MCL)"=w4864) -> ("FPGA VI Reference Out"=w4866:T24, "error out"=w4865:errorcluster)
          }
        }
        "Raster Scanning..." <- TRUE ("Scanning...")
      }
    }
    n2514 = local read "Flushing P3"() -> (w3647:bool)
    n2515 = case "Keep track of when Harvard Pump 3 is done flushing" shown="True" w3647 {
      frame False {
      }
      frame True {
        n2516 = local read "Flush rate (uL/m) P3"() -> (w4022:dbl)
        n2517 = local read "DMA Update Period (s)"() -> (w4024:dbl)
        n2518 = local read "HP3 Flush Time (s)"() -> (w4031:dbl)
        n2519 = Divide(x=w4022, y=60.0) -> (x/y=w4020:dbl)
        n2520 = feedback #5(0) -> (w4029:i32)
        n2521 = Increment(x=w4029) -> (x+1=w4023:i32)
        n2522 = Divide(x=w4031, y=w4024) -> (x/y=w4025:dbl)
        n2523 = Greater?(x=w4023, y=w4025) -> (0:w4028:bool)
        n2524 = Compound Arithmetic op=MULTIPLY(w4024, w4023, w4020) -> (→"P3 Flush Volume (uL)":dbl)
        n2525 = case shown="True" w4028 {
          tunnel: w4023 -> [w4032 _]
          tunnel: [w4032 0] -> w4027
          frame False {
          }
          frame True {
            w4033 = FALSE ("Flushing P3")
            n2526 = local write "Inject Pump 3"(w4033) -> ()
            n2527 = local write "Flushing P3"(w4033) -> ()
            n2528 = property on="Clear Volume P3" class="Bool (strict)"("Val(Sgnl)"=TRUE ("Value (Signaling)")) -> ()  [unwired: 2 in, 2 out]
          }
        }
        n2529 = feedback-in #5(w4027) -> ()
        n2530 = Divide(x=w4023, y=w4025) -> (x/y=→"P3 Flushing Bar":dbl)
      }
    }
    n2531 = And(x="Save scans", y=w3846) -> (x .and. y?=w3878:bool)
    n2532 = Compound Arithmetic op=OR("Start MCL Scan", "Confocal Image", "Confocal Linescan") -> (w3844:bool)
    n2533 = And(x="Save Data (MCL)", y=w3844) -> (x .and. y?=w3877:bool)
    n2534 = case "Start MCL raster scan" shown="True" w3844 {
      tunnel: w3880 -> [w4432 w4448]
      tunnel: w3879 -> [w4431 w4447]
      tunnel: [w4432 w4443] -> w3770
      tunnel: [w4431 w4442] -> w3769
      tunnel: [FALSE w4441] -> w3863
      tunnel: "Start MCL Scan" -> [_ w4436]
      tunnel: "Confocal Image" -> [_ w4435]
      tunnel: "Confocal Linescan" -> [_ _]
      frame False {
      }
      frame True {
        w4441 = TRUE
        n2535 = case shown="True" "Restart DMA? (MCL)" {